vi "Main.vi"() -> ()   [LabVIEW 2020] (continued)
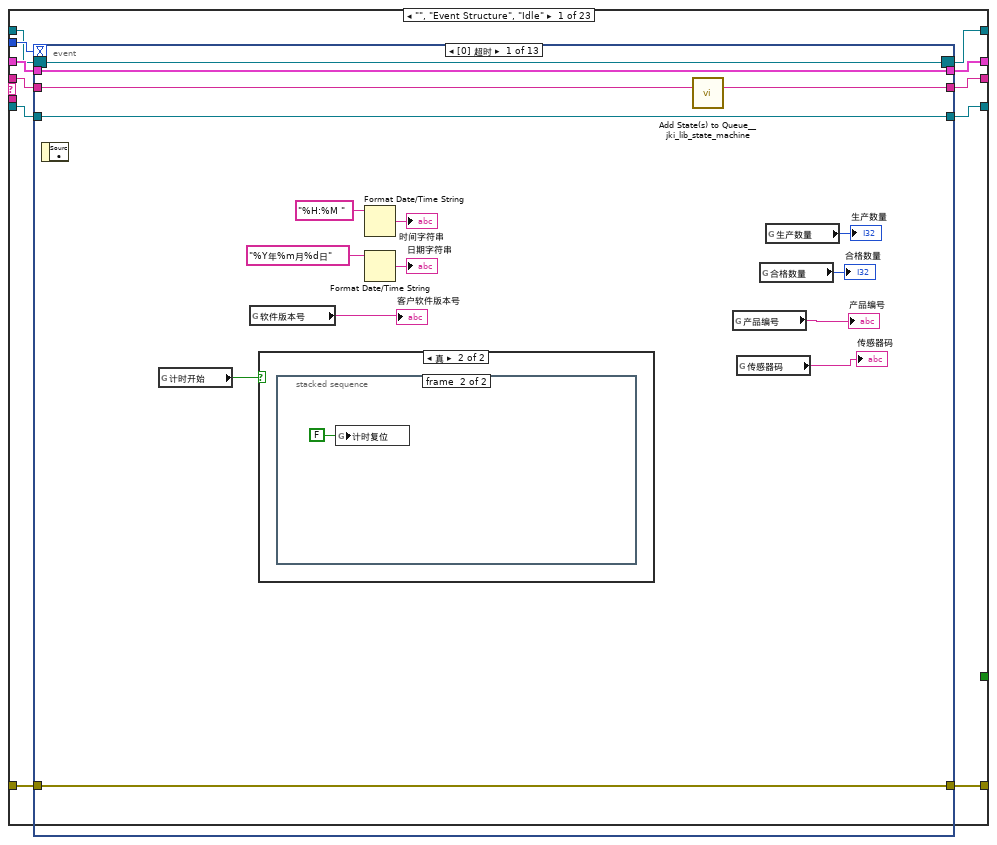
[diagram p2: hidden frame]
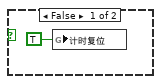
[diagram p3: hidden frame]
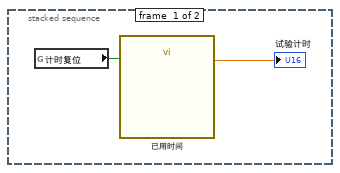
[diagram p4: hidden frame]
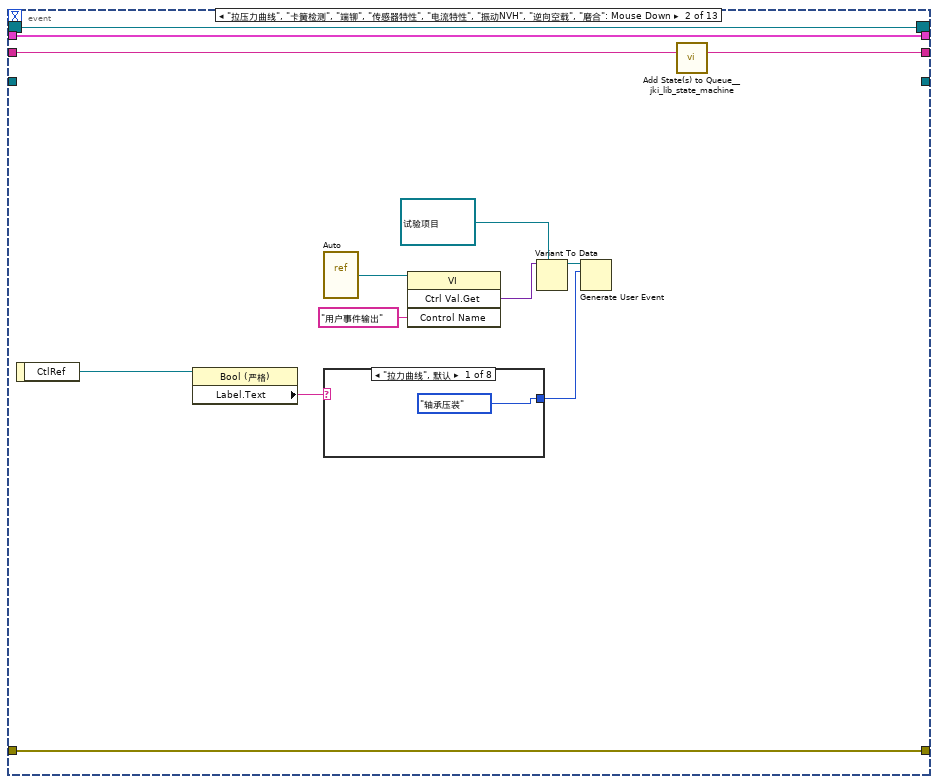
[diagram p5: hidden frame]
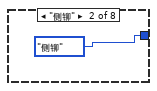
[diagram p6: hidden frame]
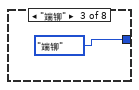
[diagram p7: hidden frame]
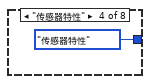
[diagram p8: hidden frame]
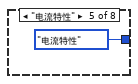
[diagram p9: hidden frame]
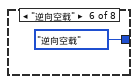
[diagram p10: hidden frame]
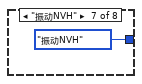
[diagram p11: hidden frame]
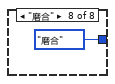
[diagram p12: hidden frame]
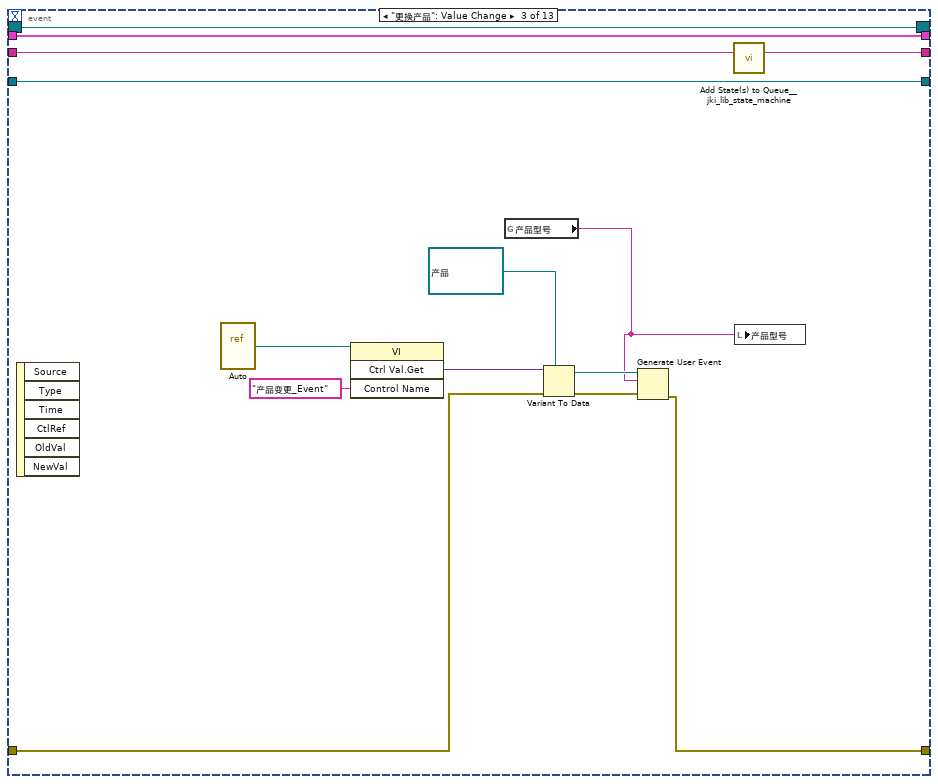
[diagram p13: hidden frame]
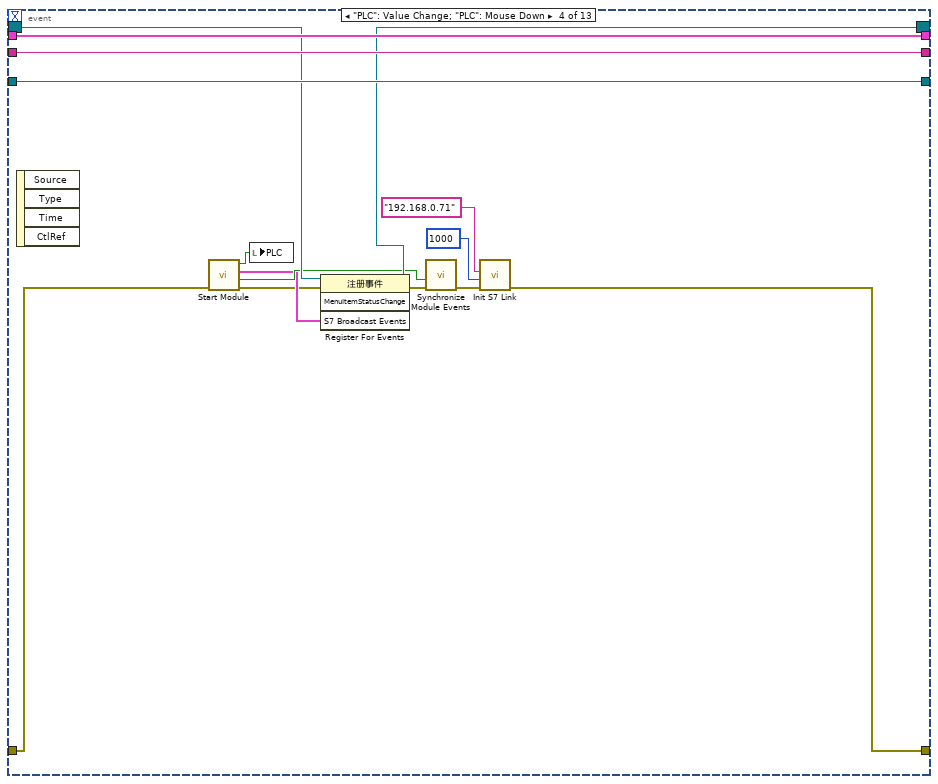
[diagram p14: hidden frame]
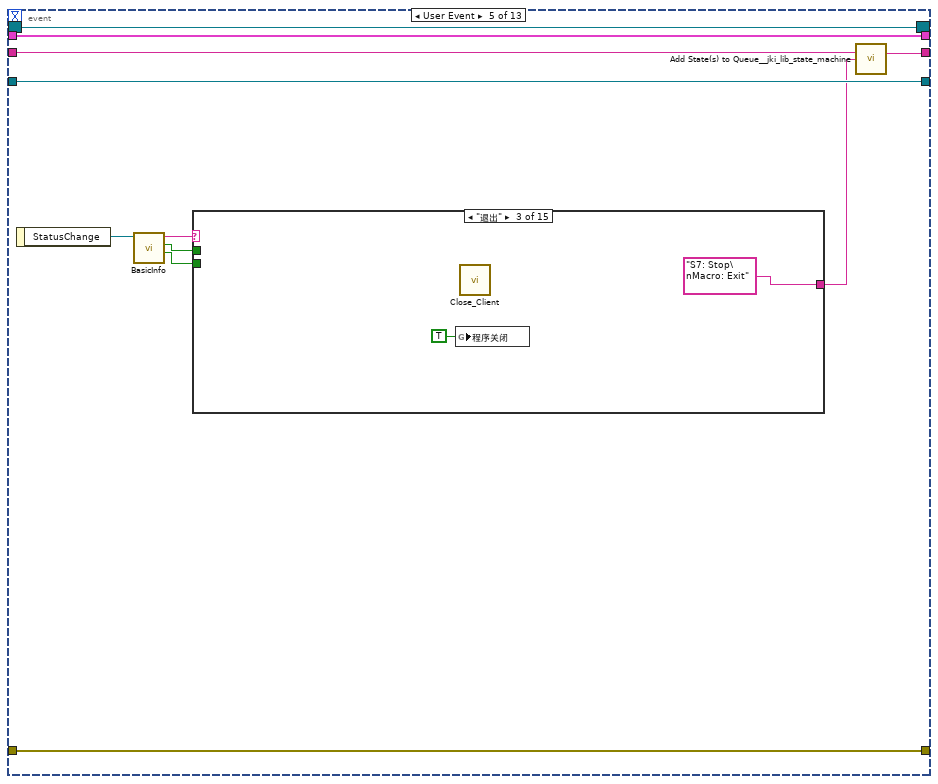
[diagram p15: hidden frame]
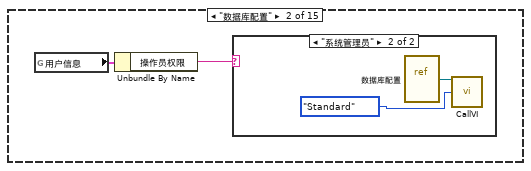
[diagram p17: hidden frame]
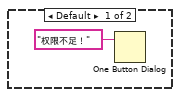
[diagram p18: hidden frame]
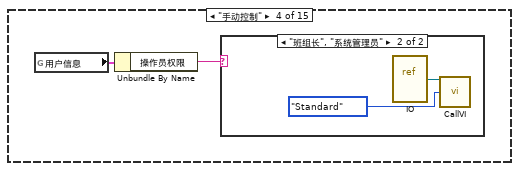
[diagram p19: hidden frame]
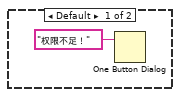
[diagram p20: hidden frame]
          }
          event "自动": Mouse Down {
            n119 = event-data() -> ()  [unwired: 1 in, 1 out]
            n120 = disable-structure shown="禁用" {
              frame Disabled {
                n121 = local read "自动"() -> (w209:bool)
                n122 = case shown="真" w209 {
                  frame False {
                    n123 = call "设备状态.vi"() -> ("Status_Read"=w210:i16)  [unwired: 11 in]
                    n124 = case shown="5" w210 {
                      frame 0, Default {
                        n125 = One Button Dialog(message="请复位！" ("消息")) -> ()  [unwired: 1 in, 1 out]
                      }
                      frame 5 {
                        n126 = vi-ref "Auto.vi"() -> (w214:refnum<vi>)
                        n127 = invoke class="VI" method="Ctrl Val.Set"(reference=w214, "Control Name"="STEP" ("控件名"), "Value"="进入自动" ("控件名")) -> ()  [unwired: 2 in, 5 out]
                      }
                    }
                  }
                  frame True {
                    n128 = Two Button Dialog(message="确定要退出自动？" ("消息")) -> (T button?=w215:bool)  [unwired: 2 in]
                    n129 = case shown="真" w215 {
                      frame False {
                      }
                      frame True {
                        n130 = vi-ref "Auto.vi"() -> (w219:refnum<vi>)
                        n131 = invoke class="VI" method="Ctrl Val.Set"(reference=w219, "Control Name"="STEP" ("控件名"), "Value"="退出自动" ("控件名")) -> ()  [unwired: 2 in, 5 out]
                      }
                    }
                  }
                }
              }
              frame Enabled {
              }
            }
            n132 = call <vilib>:"Add State(s) to Queue__jki_lib_state_machine.vi"("State(s) in (\"\")"=w205) -> ("States Out"=w206:string)  [unwired: 14 in]
          }
          event "错误": Mouse Down {
            n133 = event-data() -> ()  [unwired: 1 in, 8 out]
            n134 = vi-ref "报警信息.vi"() -> (w222:refnum<vi>)
            n135 = call "CallVI.vi"("VI引用"=w222, "状态"=T4."Standard") -> ()  [unwired: 12 in, 2 out]
            n136 = call <vilib>:"Add State(s) to Queue__jki_lib_state_machine.vi"("State(s) in (\"\")"=w224) -> ("States Out"=w225:string)  [unwired: 14 in]
          }
          event Panel Close? {
            n137 = event-data() -> ()  [unwired: 1 in, 1 out]
            n138 = global write "Global.vi" "程序关闭"(TRUE ("程序关闭")) -> ()
            n139 = call <vilib>:"Add State(s) to Queue__jki_lib_state_machine.vi"("State(s) in Front (\"\")"="S7: Stop\nMacro: Exit", "State(s) in (\"\")"=w234) -> ("States Out"=w233:string)  [unwired: 13 in]
            n140 = event-data("Discard?"=TRUE) -> ()  [unwired: 1 in, 1 out]
          }
          event "Andon": Value Change {
            n141 = event-data() -> ("NewVal"=w239:enum32{"未选择", "缺料报警", "质量报警", "故障报警"})  [unwired: 1 in]
            n142 = case shown="\"未选择\", 默认" w239 {
              tunnel: [enum16{"设备离线", "设备正常", "设备缺料", "设备故障", "质量报警"}."设备正常" ("设备状态") enum16{"设备离线", "设备正常", "设备缺料", "设备故障", "质量报警"}."设备缺料" ("设备状态") enum16{"设备离线", "设备正常", "设备缺料", "设备故障", "质量报警"}."质量报警" ("设备状态") enum16{"设备离线", "设备正常", "设备缺料", "设备故障", "质量报警"}."设备故障" ("设备状态")] -> w237
              frame "未选择", Default {
              }
              frame "缺料报警" {
              }
              frame "质量报警" {
              }
              frame "故障报警" {
              }
            }
            n143 = local read "userName"() -> (w236:string)
            n144 = Bundle By Name(cluster=T5 {"设备名称"="滑移力复检", "操作人员"="", "设备状态"=enum."设备离线", "附加信息"=""} ("设备信息"), "操作人员"=w236, "设备状态"=w237) -> (w235:T5)
            n145 = call "Change_Client.vi"("设备信息"=w235) -> ()  [unwired: 10 in, 1 out]
          }
        }
      }
      frame "---------- Core ----------" {
        n146 = call <vilib>:"Add State(s) to Queue__jki_lib_state_machine.vi"("State(s) in (\"\")"=w253) -> ("States Out"=w252:string)  [unwired: 14 in]
      }
      frame Default {
        w265 = 42 items=["No error", "Argument error", "Memory is full", "Out of zone", "End of file", "File already open", "Generic file I/O error", "File not found", "File permission error", "Disk is full", "Duplicate path", "Too many files open", "System feature not enabled", "Resource file not found", "Cannot add resource", "Resource not found", "Image not found", "Image memory error", "Pen does not exist", "Config type invalid", "Config token not found", "Config parse error", "Config memory error", "Bad external code format", "Bad external code offset", "External code not present", "Null window", "Destroy window error", "Null menu", "Print aborted", "Bad print record", "Print driver error", "Windows error during printing", "Memory error during printing", "Print dialog error", "Generic print error", "Invalid device refnum", "Device not found", "Device parameter error", "Device unit error", "Cannot open device", "Device call aborted", "Generic error", "Cancelled by user", "Object ID too low", "Object ID too high", "Object not in heap", "Unknown heap", "Unknown object (invalid DefProc)", "Unknown object (DefProc not in table)", "Message out of range", "Invalid (null) method", "Unknown message", "Manager call not supported", "Bad address", "Network operation in progress", "Network operation timed out", "Connection is busy", "Network attribute not supported", "Network error", "Address in use", "System out of memory", "Connection aborted", "Connection refused", "Not connected", "Already connected", "Connection closed", "Initialization error (interapplication manager)", "Bad occurrence", "Wait on unbound occurrence handler", "Occurrence queue overflow", "Datalog type conflict", "Unused", "Unrecognized type (interapplication manager)", "Memory corrupt", "Failed to make temporary DLL", "Old CIN version", "Drag socket not found", "Failed to load drop-object", "Failed to register OLE object", "Failed to release OLE object", "Format specifier type mismatch", "Unknown format specifier", "Too few format specifiers", "Too many format specifiers", "Scan failed", "Newer CIN version", "Error converting to variant", "Runtime menu error", "Password tampered", "Variant attribute not found", "Incompatible variant data type", "Event data is not available", "Event Store is not present", "Occurrence is not found", "Event Queue is not created", "Event info is not available", "Refnum passed is NULL", "Error retrieving Class GUID", "Error retrieving CoClass GUID", "Error retrieving TypeLib GUID.", "Bad built application magic bytes.", "Specific driver is different from the specific driver associated with the Logical Name.", "There is no session opened to the class driver.", "Max Error", "MAX - Error with config objects", "MAX - Error loading configuration", "MAX - Group not supported"]
        # "Current State"
        n147 = Format Into String(format string="Software Exception: Unhandled State \"%s\"." ("message"), error in=w261, w256) -> (resulting string=w264:string, error out=w263:errorcluster)  [unwired: 1 in]
        n148 = call <vilib>:"Error Cluster From Error Code.vi"("show call chain? (False)"=TRUE, "error in (no error)"=w263, "error message (\"\")"=w264, "error code (0)"=w265) -> ("error out"=w262:errorcluster)  [unwired: 5 in]
        n149 = call <vilib>:"Add State(s) to Queue__jki_lib_state_machine.vi"("State(s) in (\"\")"=w260) -> ("States Out"=w259:string)  [unwired: 14 in]
      }
      frame "Initialize Core Data" {
        # "originally closed?"
        # "exe?"
        n150 = property class="VI"() -> ("Front Panel.Open"=w276:bool)  [unwired: 2 in, 2 out]
        n151 = property class="App"() -> ("App.Kind"=w275:T6)  [unwired: 2 in, 2 out]
        n152 = control-ref of="Current VI Reference"() -> (w269:refnum<vi>)
        n153 = Not(x=w276) -> (.not. x?=w273:bool)
        n154 = Equal?(x=w275, y=T6."Run Time System" ("Application:Kind")) -> (x = y?=w272:bool)
        n155 = Or(x=w273, y=w272) -> (x .or. y?=w270:bool)
        n156 = Bundle By Name(cluster=w271, "Core.Current VI Reference"=w269, "Core.Close Panel on Exit?"=w270) -> (w278:T8)
        n157 = call <vilib>:"Add State(s) to Queue__jki_lib_state_machine.vi"("State(s) in (\"\")"=w280) -> ("States Out"=w279:string)  [unwired: 14 in]
      }
      frame "Error Handler" {
        n158 = call <vilib>:"General Error Handler.vi"("error in (no error)"=w284) -> ()  [unwired: 10 in, 5 out]
        n159 = call <vilib>:"Add State(s) to Queue__jki_lib_state_machine.vi"("State(s) in Front (\"\")"="/* Post Error States", "State(s) in (\"\")"=w288) -> ("States Out"=w287:string)  [unwired: 13 in]
      }
      frame "Exit" {
        n160 = call <vilib>:"Add State(s) to Queue__jki_lib_state_machine.vi"("State(s) in (\"\")"=w295) -> ("States Out"=w294:string)  [unwired: 14 in]
        n161 = Quit LabVIEW() -> ()  [unwired: 1 in]
      }
      frame "--------- Library --------" {
        n162 = call <vilib>:"Add State(s) to Queue__jki_lib_state_machine.vi"("State(s) in (\"\")"=w301) -> ("States Out"=w300:string)  [unwired: 14 in]
      }
      frame "S7: Initialize" {
        n163 = property on="PLC" class="Bool (严格)"("Val(Sgnl)"=FALSE ("值(信号)")) -> ()  [unwired: 2 in, 2 out]
      }
      frame "S7: Stop" {
        n164 = call "Stop Module.vi"("error in (no error)"=w310) -> ("error out"=w309:errorcluster)  [unwired: 10 in]
        n165 = call <vilib>:"Add State(s) to Queue__jki_lib_state_machine.vi"("State(s) in (\"\")"=w311) -> ("States Out"=w312:string)  [unwired: 14 in]
      }
      frame "CAN: Start" {
        n166 = call <vilib>:"Add State(s) to Queue__jki_lib_state_machine.vi"("State(s) in (\"\")"=w317) -> ("States Out"=w318:string)  [unwired: 14 in]
      }
      frame "CAN: Stop" {
        n167 = call <vilib>:"Add State(s) to Queue__jki_lib_state_machine.vi"("State(s) in (\"\")"=w323) -> ("States Out"=w324:string)  [unwired: 14 in]
      }
      frame "---------- Data ----------" {
        n168 = call <vilib>:"Add State(s) to Queue__jki_lib_state_machine.vi"("State(s) in (\"\")"=w332) -> ("States Out"=w331:string)  [unwired: 14 in]
      }
      frame "Data: Initialize" {
        w337 = T9 {"Current VI Reference"=refnum, "Close Panel on Exit?"=FALSE}  # Core
        w339 = TRUE  # Your Boolean data
        w338 = ""  # Your string data
        n169 = global write "Global.vi" "程序关闭"(FALSE ("程序关闭")) -> ()
        n170 = global write "Global.vi" "计时开始"(FALSE ("计时结束")) -> ()
        n171 = Bundle("Core"=w337, "Your Boolean data"=w339, "Your string data"=w338) -> (w341:T8)  [unwired: 1 in]
        n172 = call <vilib>:"Add State(s) to Queue__jki_lib_state_machine.vi"("State(s) in (\"\")"=w343) -> ("States Out"=w342:string)  [unwired: 14 in]
      }
      frame "Data: Cleanup" {
        n173 = Unbundle By Name(w346) -> ("Core.Current VI Reference"=w349:refnum<vi>)
        n174 = Close Reference(reference=w349, error in (no error)=w348) -> (error out=w347:errorcluster)
        n175 = call <vilib>:"Add State(s) to Queue__jki_lib_state_machine.vi"("State(s) in (\"\")"=w351) -> ("States Out"=w350:string)  [unwired: 14 in]
      }
      frame "---------- UI ----------" {
        # "Do not put any code in this frame.\n(It is a separator no-op. You can make a copy of this frame to create a new UI frame)"
        n176 = call <vilib>:"Add State(s) to Queue__jki_lib_state_machine.vi"("State(s) in (\"\")"=w357) -> ("States Out"=w356:string)  [unwired: 14 in]
      }
      frame "UI: Initialize" {
        n177 = disable-structure shown="启用" {
          disable-tunnel: [w373 _] -> w362
          disable-tunnel: w358 -> [w371 _]
          frame Enabled {
            n178 = vi-ref "Auto.vi"() -> (w372:refnum<vi>)
            n179 = invoke on="子面板" class="SubPnl" method="Insert VI"(error in=w371, "VI Ref"=w372) -> (error out=w376:errorcluster)  [unwired: 2 in, 3 out]
            n180 = invoke class="VI" method="Run VI"(reference=w372, error in=w376, "Wait until done"=FALSE ("结束前等待"), "Auto Dispose Ref"=TRUE ("自动销毁引用")) -> (error out=w373:errorcluster)  [unwired: 1 in, 4 out]
          }
          frame Disabled {
            n181 = vi-ref "Auto.vi"() -> (w378:refnum<vi>)
            n182 = call "CallVI.vi"("VI引用"=w378, "状态"=T4."Maximized") -> ()  [unwired: 12 in, 2 out]
          }
        }
        n183 = vi-ref "Auto_Step.vi"() -> (w359:refnum<vi>)
        n184 = invoke on="子面板" class="SubPnl" method="Insert VI"(error in=w358, "VI Ref"=w359) -> (error out=w360:errorcluster)  [unwired: 2 in, 3 out]
        n185 = invoke class="VI" method="Run VI"(reference=w359, error in=w360, "Wait until done"=FALSE ("结束前等待"), "Auto Dispose Ref"=TRUE ("自动销毁引用")) -> (error out=w363:errorcluster)  [unwired: 1 in, 4 out]
        n186 = call <vilib>:"Add State(s) to Queue__jki_lib_state_machine.vi"("State(s) in (\"\")"=w370) -> ("States Out"=w369:string)  [unwired: 14 in]
        n187 = Merge Errors(w362, w363) -> (w361:errorcluster)
      }
      frame "UI: Init" {
        n188 = stacked-sequence {
          tunnel: w380 -> [_ _ _ _]
          frame #0 {
            n189 = global write "Global.vi" "程序关闭"(FALSE ("程序关闭")) -> ()
            n190 = control-ref of="拉压力曲线"() -> (w391:refnum<vi>)
            n191 = control-ref of="电流特性"() -> (w388:refnum<vi>)
            n192 = control-ref of="端铆"() -> (w389:refnum<vi>)
            n193 = control-ref of="卡簧检测"() -> (w390:refnum<vi>)
            n194 = global write "A180648.vi" "LED-轴承压装"(w391) -> ()
            n195 = global write "A180648.vi" "LED-电流特性"(w388) -> ()
            n196 = global write "A180648.vi" "LED-侧铆"(w390) -> ()
            n197 = global write "A180648.vi" "LED-端铆"(w389) -> ()
            n198 = control-ref of="逆向空载"() -> (w387:refnum<vi>)
            n199 = control-ref of="振动NVH"() -> (w385:refnum<vi>)
            n200 = control-ref of="传感器特性"() -> (w386:refnum<vi>)
            n201 = global write "A180648.vi" "LED-传感器特性"(w386) -> ()
            n202 = global write "A180648.vi" "LED-逆向空载"(w387) -> ()
            n203 = global write "A180648.vi" "LED-振动NVH"(w385) -> ()
          }
          frame #1 {
            w398 = 0
            n204 = shared-variable "我的电脑\\Global.lvlib\\总成追溯码"("   " ("工位追溯码")) -> ()  [unwired: 1 in, 1 out]
            n205 = global write "Global.vi" "生产数量"(w398) -> ()
            n206 = global write "Global.vi" "合格数量"(w398) -> ()
            n207 = global read "Global.vi" "用户信息"() -> (w396:T10)
            n208 = global read "Global.vi" "联机模式"() -> (w393:enum16{"单机", "追溯"})
            n209 = Unbundle By Name(w396) -> ("用户名"=→"userName":string, "用户权限"=→"userStatus":string)
            n210 = case shown="\"追溯\"" w393 {
              tunnel: ["联网" ("connectionMode") "单机" ("connectionMode")] -> w399
              frame "追溯" {
              }
              frame "单机", Default {
              }
            }
            "connectionMode" <- w399
          }
          frame #2 {
            n211 = control-ref of="更换产品"() -> (w403:refnum<vi>)
            n212 = control-ref of="提示信息"() -> (w405:refnum<vi>)
            n213 = control-ref of="自动"() -> (w406:refnum<vi>)
            n214 = control-ref of="错误"() -> (w407:refnum<vi>)
            n215 = control-ref of="Result"() -> (w408:refnum<vi>)
            n216 = global write "Global.vi" "提示信息"(w405) -> ()
            n217 = global write "Global.vi" "程序自动"(w406) -> ()
            n218 = global write "Global.vi" "报警图标"(w407) -> ()
            n219 = global write "Global.vi" "Result"(w408) -> ()
            n220 = global write "Global.vi" "更改标尺"(w403) -> ()
            n221 = control-ref of="状态"() -> (w404:refnum<vi>)
            n222 = global write "Global.vi" "状态"(w404) -> ()
            "产品型号" <- "" ("产品型号")
          }
          frame #3 {
            n223 = global read "Global.vi" "Result"() -> (w411:refnum<vi>)
            n224 = property class="Tbl"(reference=w411, "Row Headers[]"=string[] [], "Value"=string[][] []) -> ()  [unwired: 1 in, 2 out]
            n225 = call "Start_Client.vi"() -> ()  [unwired: 12 in]
          }
        }
        n226 = call <vilib>:"Add State(s) to Queue__jki_lib_state_machine.vi"("State(s) in (\"\")"=w384) -> ("States Out"=w383:string)  [unwired: 14 in]
      }
      frame "UI: Config" {
        n227 = vi-ref "Config.vi"() -> (w414:refnum<vi>)
        n228 = call "CallVI.vi"("VI引用"=w414, "状态"=T4."Standard") -> ()  [unwired: 12 in, 2 out]
        n229 = call <vilib>:"Add State(s) to Queue__jki_lib_state_machine.vi"("State(s) in (\"\")"=w419) -> ("States Out"=w418:string)  [unwired: 14 in]
      }
      frame "UI: Cursor Set" {
        # "Argument"
        n230 = case shown="\"Idle\", 默认" w422 {
          tunnel: w424 -> [w429 w431]
          tunnel: [w428 w430] -> w423
          frame "Idle", Default {
            n231 = call <vilib>:"Unset Busy.vi"("error in (no error)"=w429) -> ("error out"=w428:errorcluster)  [unwired: 10 in]
          }
          frame "Busy" {
            n232 = call <vilib>:"Set Busy.vi"("error in (no error)"=w431) -> ("error out"=w430:errorcluster)  [unwired: 9 in, 1 out]
          }
        }
        n233 = call <vilib>:"Add State(s) to Queue__jki_lib_state_machine.vi"("State(s) in (\"\")"=w427) -> ("States Out"=w426:string)  [unwired: 14 in]
      }
      frame "UI: Front Panel State" {
        # "Argument"
        n234 = Unbundle By Name(w436) -> ("Core.Current VI Reference"=w435:refnum<vi>)
        n235 = case shown="\"Close\"" w434 {
          tunnel: w438 -> [w444 w457]
          tunnel: [w446 w458] -> w437
          tunnel: w435 -> [w445 w455]
          frame "Open", Default {
            n236 = property class="VI"(reference=w445, error in=w444) -> (reference out=w442:refnum<vi>, error out=w443:errorcluster, "Front Panel.Open"=w441:bool)
            n237 = case shown="假" w441 {
              tunnel: [w449 w452] -> w446
              tunnel: w443 -> [w448 w452]
              tunnel: w442 -> [w447 _]
              frame False {
                n238 = invoke class="VI" method="FP.Open"(reference=w447, error in=w448, "Activate"=TRUE, "State"=T4."Standard") -> (error out=w449:errorcluster)  [unwired: 1 in, 4 out]
              }
              frame True {
              }
            }
          }
          frame "Close" {
            n239 = property class="VI"(reference=w455, error in=w457) -> (reference out=w454:refnum<vi>, error out=w456:errorcluster, "Front Panel.Open"=w453:bool)
            n240 = case shown="真" w453 {
              tunnel: [w459 w462] -> w458
              tunnel: w456 -> [w459 w461]
              tunnel: w454 -> [_ w460]
              frame False {
              }
              frame True {
                n241 = invoke class="VI" method="FP.Close"(reference=w460, error in=w461) -> (error out=w462:errorcluster)  [unwired: 1 in, 2 out]
              }
            }
          }
        }
        n242 = call <vilib>:"Add State(s) to Queue__jki_lib_state_machine.vi"("State(s) in (\"\")"=w440) -> ("States Out"=w439:string)  [unwired: 14 in]
      }
      frame "---------- Macro ----------" {
        n243 = call <vilib>:"Add State(s) to Queue__jki_lib_state_machine.vi"("State(s) in (\"\")"=w468) -> ("States Out"=w467:string)  [unwired: 14 in]
      }
      frame "Macro: Initialize" {
        n244 = call <vilib>:"Add State(s) to Queue__jki_lib_state_machine.vi"("State(s) in Front (\"\")"="Data: Initialize\nInitialize Core Data\nS7: Initialize\nIdle\nUI: Init\nUI: Front Panel State >> Open\nUI: Initialize\nUI: Config", "State(s) in (\"\")"=w475) -> ("States Out"=w474:string)  [unwired: 13 in]
      }
      frame "Macro: Exit" {
        n245 = Unbundle By Name(w484) -> ("Core.Close Panel on Exit?"=w483:bool)
        n246 = Select(t="UI: Front Panel State >> Close", s=w483, f="") -> (s? t:f=w480:string)
        n247 = call <vilib>:"Add State(s) to Queue__jki_lib_state_machine.vi"("State(s) in (\"\")"=w480, "State(s) at Back (\"\")"="Data: Cleanup\nExit") -> ("States Out"=w478:string)  [unwired: 13 in]
        n248 = call <vilib>:"Add State(s) to Queue__jki_lib_state_machine.vi"("State(s) in Front (\"\")"=w478, "State(s) in (\"\")"=w487) -> ("States Out"=w486:string)  [unwired: 13 in]
      }
    }
  }
  n249 = call-dynamic "Cleanup.vi"("MenuStrip in"=w6) -> ()  [unwired: 10 in, 1 out]
